vi "SaccadeAnalyser - Main.vi"(8 "error in (no error)":errorcluster, 11 "Data IN":T3={"Impulse Positions"=[{"Start"=5471, "End"=5813, "Impulse Plane"=enum."Yaw", "Impulse Direction +ve?"=FALSE, "Time offset"=0, "Amplitude offset"=0.0}, {"Start"=6974, "End"=7325, "Impulse Plane"=enum."Yaw", "Impulse Direction +ve?"=TRUE, "Time offset"=0, "Amplitude offset"=0.0}, {"Start"=7641, "End"=7980, "Impulse Plane"=enum."Yaw", "Impulse Direction +ve?"=FALSE, "Time offset"=0, "Amplitude offset"=0.0}, {"Start"=9060, "End"=9400, "Impulse Plane"=enum."Yaw", "Impulse Direction +ve?"=FALSE, "Time offset"=0, "Amplitude offset"=0.0}, {"Start"=9938, "End"=10282, "Impulse Plane"=enum."Yaw", "Impulse Direction +ve?"=FALSE, "Time offset"=0, "Amplitude offset"=0.0}, {"Start"=10800, "End"=11142, "Impulse Plane"=enum."Yaw", "Impulse Direction +ve?"=FALSE, "Time offset"=0, "Amplitude offset"=0.0}, {"Start"=11602, "End"=11942, "Impulse Plane"=enum."Yaw", "Impulse Direction +ve?"=TRUE, "Time offset"=0, "Amplitude offset"=0.0}, {"Start"=12449, "End"=12790, "Impulse Plane"=enum."Yaw", "Impulse Direction +ve?"=TRUE, "Time offset"=0, "Amplitude offset"=0.0}, {"Start"=13310, "End"=13653, "Impulse Plane"=enum."Yaw", "Impulse Direction +ve?"=TRUE, "Time offset"=0, "Amplitude offset"=0.0}, {"Start"=14191, "End"=14535, "Impulse Plane"=enum."Yaw", "Impulse Direction +ve?"=TRUE, "Time offset"=0, "Amplitude offset"=0.0}, {"Start"=15040, "End"=15380, "Impulse Plane"=enum."Yaw", "Impulse Direction +ve?"=FALSE, "Time offset"=0, "Amplitude offset"=0.0}, {"Start"=16780, "End"=17124, "Impulse Plane"=enum."Yaw", "Impulse Direction +ve?"=TRUE, "Time offset"=0, "Amplitude offset"=0.0}, {"Start"=17572, "End"=17913, "Impulse Plane"=enum."Yaw", "Impulse Direction +ve?"=FALSE, "Time offset"=0, "Amplitude offset"=0.0}, {"Start"=18369, "End"=18713, "Impulse Plane"=enum."Yaw", "Impulse Direction +ve?"=FALSE, "Time offset"=0, "Amplitude offset"=0.0}, {"Start"=19174, "End"=19519, "Impulse Plane"=enum."Yaw", "Impulse Direction +ve?"=FALSE, "Time offset"=0, "Amplitude offset"=0.0}, {"Start"=19928, "End"=20270, "Impulse Plane"=enum."Yaw", "Impulse Direction +ve?"=TRUE, "Time offset"=0, "Amplitude offset"=0.0}, {"Start"=20762, "End"=21121, "Impulse Plane"=enum."Yaw", "Impulse Direction +ve?"=FALSE, "Time offset"=0, "Amplitude offset"=0.0}, {"Start"=21554, "End"=21888, "Impulse Plane"=enum."Yaw", "Impulse Direction +ve?"=FALSE, "Time offset"=0, "Amplitude offset"=0.0}, {"Start"=22293, "End"=22639, "Impulse Plane"=enum."Yaw", "Impulse Direction +ve?"=TRUE, "Time offset"=0, "Amplitude offset"=0.0}, {"Start"=23109, "End"=23464, "Impulse Plane"=enum."Yaw", "Impulse Direction +ve?"=TRUE, "Time offset"=0, "Amplitude offset"=0.0}, {"Start"=23868, "End"=24215, "Impulse Plane"=enum."Yaw", "Impulse Direction +ve?"=TRUE, "Time offset"=0, "Amplitude offset"=0.0}, {"Start"=24643, "End"=24992, "Impulse Plane"=enum."Yaw", "Impulse Direction +ve?"=FALSE, "Time offset"=0, "Amplitude offset"=0.0}, {"Start"=25685, "End"=26023, "Impulse Plane"=enum."Yaw", "Impulse Direction +ve?"=FALSE, "Time offset"=0, "Amplitude offset"=0.0}, {"Start"=26431, "End"=26768, "Impulse Plane"=enum."Yaw", "Impulse Direction +ve?"=FALSE, "Time offset"=0, "Amplitude offset"=0.0}, {"Start"=27251, "End"=27595, "Impulse Plane"=enum."Yaw", "Impulse Direction +ve?"=FALSE, "Time offset"=0, "Amplitude offset"=0.0}, {"Start"=28832, "End"=29180, "Impulse Plane"=enum."Yaw", "Impulse Direction +ve?"=TRUE, "Time offset"=0, "Amplitude offset"=0.0}, {"Start"=31028, "End"=31383, "Impulse Plane"=enum."LARP", "Impulse Direction +ve?"=FALSE, "Time offset"=0, "Amplitude offset"=0.0}, {"Start"=32603, "End"=32936, "Impulse Plane"=enum."LARP", "Impulse Direction +ve?"=TRUE, "Time offset"=0, "Amplitude offset"=0.0}, {"Start"=33445, "End"=33779, "Impulse Plane"=enum."LARP", "Impulse Direction +ve?"=TRUE, "Time offset"=0, "Amplitude offset"=0.0}, {"Start"=34276, "End"=34629, "Impulse Plane"=enum."LARP", "Impulse Direction +ve?"=FALSE, "Time offset"=0, "Amplitude offset"=0.0}, {"Start"=35114, "End"=35460, "Impulse Plane"=enum."LARP", "Impulse Direction +ve?"=FALSE, "Time offset"=0, "Amplitude offset"=0.0}, {"Start"=35981, "End"=36324, "Impulse Plane"=enum."LARP", "Impulse Direction +ve?"=TRUE, "Time offset"=0, "Amplitude offset"=0.0}, {"Start"=36920, "End"=37249, "Impulse Plane"=enum."LARP", "Impulse Direction +ve?"=TRUE, "Time offset"=0, "Amplitude offset"=0.0}, {"Start"=37988, "End"=38322, "Impulse Plane"=enum."LARP", "Impulse Direction +ve?"=TRUE, "Time offset"=0, "Amplitude offset"=0.0}, {"Start"=38964, "End"=39324, "Impulse Plane"=enum."LARP", "Impulse Direction +ve?"=FALSE, "Time offset"=0, "Amplitude offset"=0.0}, {"Start"=39948, "End"=40284, "Impulse Plane"=enum."LARP", "Impulse Direction +ve?"=TRUE, "Time offset"=0, "Amplitude offset"=0.0}, {"Start"=40958, "End"=41293, "Impulse Plane"=enum."LARP", "Impulse Direction +ve?"=TRUE, "Time offset"=0, "Amplitude offset"=0.0}, {"Start"=41899, "End"=42229, "Impulse Plane"=enum."LARP", "Impulse Direction +ve?"=TRUE, "Time offset"=0, "Amplitude offset"=0.0}, {"Start"=42801, "End"=43154, "Impulse Plane"=enum."LARP", "Impulse Direction +ve?"=FALSE, "Time offset"=0, "Amplitude offset"=0.0}, {"Start"=43641, "End"=43980, "Impulse Plane"=enum."LARP", "Impulse Direction +ve?"=TRUE, "Time offset"=0, "Amplitude offset"=0.0}, {"Start"=44466, "End"=44821, "Impulse Plane"=enum."LARP", "Impulse Direction +ve?"=FALSE, "Time offset"=0, "Amplitude offset"=0.0}, {"Start"=45388, "End"=45722, "Impulse Plane"=enum."LARP", "Impulse Direction +ve?"=TRUE, "Time offset"=0, "Amplitude offset"=0.0}, {"Start"=46149, "End"=46510, "Impulse Plane"=enum."LARP", "Impulse Direction +ve?"=FALSE, "Time offset"=0, "Amplitude offset"=0.0}, {"Start"=47874, "End"=48206, "Impulse Plane"=enum."LARP", "Impulse Direction +ve?"=TRUE, "Time offset"=0, "Amplitude offset"=0.0}, {"Start"=50143, "End"=50479, "Impulse Plane"=enum."RALP", "Impulse Direction +ve?"=TRUE, "Time offset"=0, "Amplitude offset"=0.0}, {"Start"=50976, "End"=51310, "Impulse Plane"=enum."RALP", "Impulse Direction +ve?"=FALSE, "Time offset"=0, "Amplitude offset"=0.0}, {"Start"=51892, "End"=52226, "Impulse Plane"=enum."RALP", "Impulse Direction +ve?"=FALSE, "Time offset"=0, "Amplitude offset"=0.0}, {"Start"=52839, "End"=53171, "Impulse Plane"=enum."RALP", "Impulse Direction +ve?"=FALSE, "Time offset"=0, "Amplitude offset"=0.0}, {"Start"=53676, "End"=54012, "Impulse Plane"=enum."RALP", "Impulse Direction +ve?"=TRUE, "Time offset"=0, "Amplitude offset"=0.0}, {"Start"=54530, "End"=54877, "Impulse Plane"=enum."RALP", "Impulse Direction +ve?"=FALSE, "Time offset"=0, "Amplitude offset"=0.0}, {"Start"=55371, "End"=55711, "Impulse Plane"=enum."RALP", "Impulse Direction +ve?"=TRUE, "Time offset"=0, "Amplitude offset"=0.0}, {"Start"=56153, "End"=56482, "Impulse Plane"=enum."RALP", "Impulse Direction +ve?"=FALSE, "Time offset"=0, "Amplitude offset"=0.0}, {"Start"=57053, "End"=57390, "Impulse Plane"=enum."RALP", "Impulse Direction +ve?"=FALSE, "Time offset"=0, "Amplitude offset"=0.0}, {"Start"=57954, "End"=58292, "Impulse Plane"=enum."RALP", "Impulse Direction +ve?"=FALSE, "Time offset"=0, "Amplitude offset"=0.0}, {"Start"=58794, "End"=59130, "Impulse Plane"=enum."RALP", "Impulse Direction +ve?"=TRUE, "Time offset"=0, "Amplitude offset"=0.0}, {"Start"=59587, "End"=59931, "Impulse Plane"=enum."RALP", "Impulse Direction +ve?"=TRUE, "Time offset"=0, "Amplitude offset"=0.0}, {"Start"=60399, "End"=60744, "Impulse Plane"=enum."RALP", "Impulse Direction +ve?"=FALSE, "Time offset"=0, "Amplitude offset"=0.0}, {"Start"=61218, "End"=61559, "Impulse Plane"=enum."RALP", "Impulse Direction +ve?"=FALSE, "Time offset"=0, "Amplitude offset"=0.0}, {"Start"=62100, "End"=62442, "Impulse Plane"=enum."RALP", "Impulse Direction +ve?"=FALSE, "Time offset"=0, "Amplitude offset"=0.0}, {"Start"=62989, "End"=63322, "Impulse Plane"=enum."RALP", "Impulse Direction +ve?"=FALSE, "Time offset"=0, "Amplitude offset"=0.0}, {"Start"=63787, "End"=64136, "Impulse Plane"=enum."RALP", "Impulse Direction +ve?"=TRUE, "Time offset"=0, "Amplitude offset"=0.0}, {"Start"=64603, "End"=64953, "Impulse Plane"=enum."RALP", "Impulse Direction +ve?"=FALSE, "Time offset"=0, "Amplitude offset"=0.0}, {"Start"=65462, "End"=65795, "Impulse Plane"=enum."RALP", "Impulse Direction +ve?"=FALSE, "Time offset"=0, "Amplitude offset"=0.0}, {"Start"=66308, "End"=66645, "Impulse Plane"=enum."RALP", "Impulse Direction +ve?"=FALSE, "Time offset"=0, "Amplitude offset"=0.0}, {"Start"=67052, "End"=67402, "Impulse Plane"=enum."RALP", "Impulse Direction +ve?"=TRUE, "Time offset"=0, "Amplitude offset"=0.0}], "No. Imp"=15, "Parameter Time Series"=[{"time offset"=0.0, "Offset"=0.0, "Gain"=1.0, "inverse"=FALSE, "filter data"=FALSE, "dots"=FALSE, "interpolate"=FALSE, "List 1"=5, "Color Box"=6618880, "Boolean"=TRUE}, {"time offset"=0.0, "Offset"=0.0, "Gain"=1.0, "inverse"=FALSE, "filter data"=FALSE, "dots"=FALSE, "interpolate"=FALSE, "List 1"=6, "Color Box"=6618880, "Boolean"=FALSE}, {"time offset"=0.0, "Offset"=0.0, "Gain"=1.0, "inverse"=FALSE, "filter data"=FALSE, "dots"=FALSE, "interpolate"=FALSE, "List 1"=7, "Color Box"=6618880, "Boolean"=FALSE}, {"time offset"=0.0, "Offset"=0.0, "Gain"=1.0, "inverse"=FALSE, "filter data"=FALSE, "dots"=FALSE, "interpolate"=FALSE, "List 1"=13, "Color Box"=16777224, "Boolean"=TRUE}, {"time offset"=0.0, "Offset"=0.0, "Gain"=1.0, "inverse"=FALSE, "filter data"=FALSE, "dots"=FALSE, "interpolate"=FALSE, "List 1"=14, "Color Box"=16777224, "Boolean"=FALSE}, {"time offset"=0.0, "Offset"=0.0, "Gain"=1.0, "inverse"=FALSE, "filter data"=FALSE, "dots"=FALSE, "interpolate"=FALSE, "List 1"=15, "Color Box"=16777224, "Boolean"=FALSE}], "Parameter Impuls Series"=[{"Color"=6618880, "Visible"=TRUE, "Channel"=1, "Invert"=FALSE, "Desaccade"=FALSE, "Offset"=0.0, "Gain"=1.0}, {"Color"=6618880, "Visible"=FALSE, "Channel"=6, "Invert"=FALSE, "Desaccade"=FALSE, "Offset"=0.0, "Gain"=1.0}, {"Color"=6618880, "Visible"=FALSE, "Channel"=7, "Invert"=FALSE, "Desaccade"=FALSE, "Offset"=0.0, "Gain"=1.0}, {"Color"=16777224, "Visible"=TRUE, "Channel"=13, "Invert"=FALSE, "Desaccade"=FALSE, "Offset"=0.0, "Gain"=1.0}, {"Color"=16777224, "Visible"=FALSE, "Channel"=14, "Invert"=FALSE, "Desaccade"=FALSE, "Offset"=0.0, "Gain"=1.0}, {"Color"=16777224, "Visible"=FALSE, "Channel"=15, "Invert"=FALSE, "Desaccade"=FALSE, "Offset"=0.0, "Gain"=1.0}], "Experiment Parameters"={"Freq"=0.0, "Vel"=0, "Acc"=0, "Stimulus"="Head Impulse"}, "Autosort File"=refnum, "Data File"={"Data Channels"=array34x71049[2415666 elements], "Sample Rate"=500, "Channel List"=["Hz Position-in-Head", "Hz Velocity-in-Head", "Hy Position-in-Head", "Hy Velocity-in-Head", "Hx Position-in-Head", "Hx Velocity-in-Head", "Hl Velocity-in-Head", "Hr Velocity-in-Head", "Lx Position-in-Head", "Ly Position-in-Head", "Lz Position-in-Head", "Lx Velocity-in-Head", "Ly Velocity-in-Head", "Lz Velocity-in-Head", "Ll Velocity-in-Head", "Lr Velocity-in-Head", "Rx Position-in-Head", "Ry Position-in-Head", "Rz Position-in-Head", "Rx Velocity-in-Head", "Ry Velocity-in-Head", "Rz Velocity-in-Head", "Rl Velocity-in-Head", "Rr Velocity-in-Head", "Target on/off", "aux input 1", "aux input 2", " ", "", "", "", "Target Hor", "Target Ver", ""]}, "Experiment data path"=path "C:/Users/w.figtree/Desktop/Coils Data/3", "Image data path"=path "/Macintosh HD/Users/patrick/Studium/Diploma Thesis/Data Analysis", "LVS data path"=path "/Macintosh HD/Users/patrick/Studium/Diploma Thesis/Data Analysis", "Raw copy path"=path "/Macintosh HD/Users/patrick/Studium/Diploma Thesis/Data Analysis", "filename"="passive_lvs.lvs", "desaccading parameters"={"Tolerance"=3, "Acc Range"=7000.0, "Sample Rate"=500, "Impulse Plane 2"=enum."Yaw", "Impulse dir"=FALSE}, "Experiment Parameters 2"={"Subject"="SE Trial Short Term", "Strain"="", "Rotation plane"="", "Experimenter"=" ", "Trial"=0.0, "Time"=0.0}, "Excel"={"Excel._Application"=refnum, "Use Excel"=TRUE, "Worksheet SINE"=refnum, "Row SINE"=0, "Worksheet TRANS"=refnum, "Row TRANS"=0}, "Session Config File"=refnum, "Autosort Parameter Set"=4, "EMA Version"="EMA 2016a", "desacc "={"Threshold 1 [Acc]"=7000.0, "Threshold 2 [% of TH1]"=60, "tolerance"=3, "Search WD "=0.1, " always use TH2"=FALSE, "Range"=3.0, "Max time"=120.0, "Min time"=20.0, "Velocity Threshold"=150}, "Cycle Nr for Saccades"={"POS"=0, "NEG"=0}, "calibration name"="u_calibration_1_p00001s001_calib.mat", "Excel"=refnum} {"Parameter Time Series"."time offset" format="%.3f"; "Parameter Time Series"."Gain" format="%.1f"; "Parameter Time Series"."Offset" format="%.1f"; "Parameter Time Series"."List 1" items=["Motor-Pos", "Motor-Vel", "Lx Position-in-Head", "Ly Position-in-Head", "Lz Position-in-Head", "Lx Velocity-in-Head", "Ly Velocity-in-Head", "Lz Velocity-in-Head", "Ll Velocity-in-Head", "Lr Velocity-in-Head", "Lx Accel-in-Head", "Ly Accel-in-Head", "Lz Accel-in-Head", "Rx Position-in-Head", "Ry Position-in-Head", "Rz Position-in-Head", "Rx Velocity-in-Head", "Ry Velocity-in-Head", "Rz Velocity-in-Head", "Rl Velocity-in-Head", "Rr Velocity-in-Head", "Rx Accel-in-Head", "Ry Accel-in-Head", "Rz Accel-in-Head", "Global Trigger", "", "", ""]; "Parameter Impuls Series"."Gain" format="%.1f"; "Parameter Impuls Series"."Offset" format="%.1f"}) -> (0 "error out":errorcluster, 3 "Data OUT":T3={"Impulse Positions"=[{"Start"=5471, "End"=5813, "Impulse Plane"=enum."Yaw", "Impulse Direction +ve?"=FALSE, "Time offset"=0, "Amplitude offset"=0.0}, {"Start"=6974, "End"=7325, "Impulse Plane"=enum."Yaw", "Impulse Direction +ve?"=TRUE, "Time offset"=0, "Amplitude offset"=0.0}, {"Start"=7641, "End"=7980, "Impulse Plane"=enum."Yaw", "Impulse Direction +ve?"=FALSE, "Time offset"=0, "Amplitude offset"=0.0}, {"Start"=9060, "End"=9400, "Impulse Plane"=enum."Yaw", "Impulse Direction +ve?"=FALSE, "Time offset"=0, "Amplitude offset"=0.0}, {"Start"=9938, "End"=10282, "Impulse Plane"=enum."Yaw", "Impulse Direction +ve?"=FALSE, "Time offset"=0, "Amplitude offset"=0.0}, {"Start"=10800, "End"=11142, "Impulse Plane"=enum."Yaw", "Impulse Direction +ve?"=FALSE, "Time offset"=0, "Amplitude offset"=0.0}, {"Start"=11602, "End"=11942, "Impulse Plane"=enum."Yaw", "Impulse Direction +ve?"=TRUE, "Time offset"=0, "Amplitude offset"=0.0}, {"Start"=12449, "End"=12790, "Impulse Plane"=enum."Yaw", "Impulse Direction +ve?"=TRUE, "Time offset"=0, "Amplitude offset"=0.0}, {"Start"=13310, "End"=13653, "Impulse Plane"=enum."Yaw", "Impulse Direction +ve?"=TRUE, "Time offset"=0, "Amplitude offset"=0.0}, {"Start"=14191, "End"=14535, "Impulse Plane"=enum."Yaw", "Impulse Direction +ve?"=TRUE, "Time offset"=0, "Amplitude offset"=0.0}, {"Start"=15040, "End"=15380, "Impulse Plane"=enum."Yaw", "Impulse Direction +ve?"=FALSE, "Time offset"=0, "Amplitude offset"=0.0}, {"Start"=16780, "End"=17124, "Impulse Plane"=enum."Yaw", "Impulse Direction +ve?"=TRUE, "Time offset"=0, "Amplitude offset"=0.0}, {"Start"=17572, "End"=17913, "Impulse Plane"=enum."Yaw", "Impulse Direction +ve?"=FALSE, "Time offset"=0, "Amplitude offset"=0.0}, {"Start"=18369, "End"=18713, "Impulse Plane"=enum."Yaw", "Impulse Direction +ve?"=FALSE, "Time offset"=0, "Amplitude offset"=0.0}, {"Start"=19174, "End"=19519, "Impulse Plane"=enum."Yaw", "Impulse Direction +ve?"=FALSE, "Time offset"=0, "Amplitude offset"=0.0}, {"Start"=19928, "End"=20270, "Impulse Plane"=enum."Yaw", "Impulse Direction +ve?"=TRUE, "Time offset"=0, "Amplitude offset"=0.0}, {"Start"=20762, "End"=21121, "Impulse Plane"=enum."Yaw", "Impulse Direction +ve?"=FALSE, "Time offset"=0, "Amplitude offset"=0.0}, {"Start"=21554, "End"=21888, "Impulse Plane"=enum."Yaw", "Impulse Direction +ve?"=FALSE, "Time offset"=0, "Amplitude offset"=0.0}, {"Start"=22293, "End"=22639, "Impulse Plane"=enum."Yaw", "Impulse Direction +ve?"=TRUE, "Time offset"=0, "Amplitude offset"=0.0}, {"Start"=23109, "End"=23464, "Impulse Plane"=enum."Yaw", "Impulse Direction +ve?"=TRUE, "Time offset"=0, "Amplitude offset"=0.0}, {"Start"=23868, "End"=24215, "Impulse Plane"=enum."Yaw", "Impulse Direction +ve?"=TRUE, "Time offset"=0, "Amplitude offset"=0.0}, {"Start"=24643, "End"=24992, "Impulse Plane"=enum."Yaw", "Impulse Direction +ve?"=FALSE, "Time offset"=0, "Amplitude offset"=0.0}, {"Start"=25685, "End"=26023, "Impulse Plane"=enum."Yaw", "Impulse Direction +ve?"=FALSE, "Time offset"=0, "Amplitude offset"=0.0}, {"Start"=26431, "End"=26768, "Impulse Plane"=enum."Yaw", "Impulse Direction +ve?"=FALSE, "Time offset"=0, "Amplitude offset"=0.0}, {"Start"=27251, "End"=27595, "Impulse Plane"=enum."Yaw", "Impulse Direction +ve?"=FALSE, "Time offset"=0, "Amplitude offset"=0.0}, {"Start"=28832, "End"=29180, "Impulse Plane"=enum."Yaw", "Impulse Direction +ve?"=TRUE, "Time offset"=0, "Amplitude offset"=0.0}, {"Start"=31028, "End"=31383, "Impulse Plane"=enum."LARP", "Impulse Direction +ve?"=FALSE, "Time offset"=0, "Amplitude offset"=0.0}, {"Start"=32603, "End"=32936, "Impulse Plane"=enum."LARP", "Impulse Direction +ve?"=TRUE, "Time offset"=0, "Amplitude offset"=0.0}, {"Start"=33445, "End"=33779, "Impulse Plane"=enum."LARP", "Impulse Direction +ve?"=TRUE, "Time offset"=0, "Amplitude offset"=0.0}, {"Start"=34276, "End"=34629, "Impulse Plane"=enum."LARP", "Impulse Direction +ve?"=FALSE, "Time offset"=0, "Amplitude offset"=0.0}, {"Start"=35114, "End"=35460, "Impulse Plane"=enum."LARP", "Impulse Direction +ve?"=FALSE, "Time offset"=0, "Amplitude offset"=0.0}, {"Start"=35981, "End"=36324, "Impulse Plane"=enum."LARP", "Impulse Direction +ve?"=TRUE, "Time offset"=0, "Amplitude offset"=0.0}, {"Start"=36920, "End"=37249, "Impulse Plane"=enum."LARP", "Impulse Direction +ve?"=TRUE, "Time offset"=0, "Amplitude offset"=0.0}, {"Start"=37988, "End"=38322, "Impulse Plane"=enum."LARP", "Impulse Direction +ve?"=TRUE, "Time offset"=0, "Amplitude offset"=0.0}, {"Start"=38964, "End"=39324, "Impulse Plane"=enum."LARP", "Impulse Direction +ve?"=FALSE, "Time offset"=0, "Amplitude offset"=0.0}, {"Start"=39948, "End"=40284, "Impulse Plane"=enum."LARP", "Impulse Direction +ve?"=TRUE, "Time offset"=0, "Amplitude offset"=0.0}, {"Start"=40958, "End"=41293, "Impulse Plane"=enum."LARP", "Impulse Direction +ve?"=TRUE, "Time offset"=0, "Amplitude offset"=0.0}, {"Start"=41899, "End"=42229, "Impulse Plane"=enum."LARP", "Impulse Direction +ve?"=TRUE, "Time offset"=0, "Amplitude offset"=0.0}, {"Start"=42801, "End"=43154, "Impulse Plane"=enum."LARP", "Impulse Direction +ve?"=FALSE, "Time offset"=0, "Amplitude offset"=0.0}, {"Start"=43641, "End"=43980, "Impulse Plane"=enum."LARP", "Impulse Direction +ve?"=TRUE, "Time offset"=0, "Amplitude offset"=0.0}, {"Start"=44466, "End"=44821, "Impulse Plane"=enum."LARP", "Impulse Direction +ve?"=FALSE, "Time offset"=0, "Amplitude offset"=0.0}, {"Start"=45388, "End"=45722, "Impulse Plane"=enum."LARP", "Impulse Direction +ve?"=TRUE, "Time offset"=0, "Amplitude offset"=0.0}, {"Start"=46149, "End"=46510, "Impulse Plane"=enum."LARP", "Impulse Direction +ve?"=FALSE, "Time offset"=0, "Amplitude offset"=0.0}, {"Start"=47874, "End"=48206, "Impulse Plane"=enum."LARP", "Impulse Direction +ve?"=TRUE, "Time offset"=0, "Amplitude offset"=0.0}, {"Start"=50143, "End"=50479, "Impulse Plane"=enum."RALP", "Impulse Direction +ve?"=TRUE, "Time offset"=0, "Amplitude offset"=0.0}, {"Start"=50976, "End"=51310, "Impulse Plane"=enum."RALP", "Impulse Direction +ve?"=FALSE, "Time offset"=0, "Amplitude offset"=0.0}, {"Start"=51892, "End"=52226, "Impulse Plane"=enum."RALP", "Impulse Direction +ve?"=FALSE, "Time offset"=0, "Amplitude offset"=0.0}, {"Start"=52839, "End"=53171, "Impulse Plane"=enum."RALP", "Impulse Direction +ve?"=FALSE, "Time offset"=0, "Amplitude offset"=0.0}, {"Start"=53676, "End"=54012, "Impulse Plane"=enum."RALP", "Impulse Direction +ve?"=TRUE, "Time offset"=0, "Amplitude offset"=0.0}, {"Start"=54530, "End"=54877, "Impulse Plane"=enum."RALP", "Impulse Direction +ve?"=FALSE, "Time offset"=0, "Amplitude offset"=0.0}, {"Start"=55371, "End"=55711, "Impulse Plane"=enum."RALP", "Impulse Direction +ve?"=TRUE, "Time offset"=0, "Amplitude offset"=0.0}, {"Start" (continued)
52.608407400318306, 68.06098679809003, 80.42943215585183, 88.0864760597265, 89.99891509546197, 85.90799751985459, 76.36544752990858, 62.62091186359373, 46.38143453236263, 29.50492183788016, 13.707859867290857, 0.3310928457604554, -9.810012583460072, -16.45442202598098, -19.82247119153461, -20.483452553608764, -19.193953324369854, -16.74774940350339, -13.849446600754366, -11.037569111752362, -8.669405751207828, -6.917292102316395, -5.789797050590641, -5.190164981316045, -4.962518505347841, -4.93187469016212, -4.9320919709982025, -4.837167605556909, -4.587847044554708, -4.179208179540813, -3.659763768094379, -3.1208090278845084, -2.653103860344153, -2.3271525568125213, -2.1861172612544255, -2.233842916743079, -2.446189563900692, -2.777356551203642, -3.1729115127205407, -3.593585048501322, -4.014858546360711, -4.426484406643328, -4.830051913071344, -5.225505364127684, -5.604699028522771, -5.955284071910426, -6.265984392521009, -6.532840549008947, -6.76267990262583, -6.974346991783459, -7.191231058870271, -7.441351509284662, -7.752342029197125, -8.138375237447635, -8.601195262840081, -9.123078516960476, -9.673239943518213, -10.219145635835941, -10.716542542217685, -11.114227594642026, -11.370082247719761, -11.451375205364059, -11.348722192681933, -11.089585339730856, -10.727486236031975, -10.343142553232035, -10.037654243821347, -9.907641710473694, -10.028124243024223, -10.440559585131421, -11.147679111533204, -12.104742918852578, -13.216616186504224, -14.363595848676741, -15.431203656896052, -16.31897411242039, -16.94639318528374, -17.271721118269923, -17.301470159658848, -17.08278383403612, -16.6966662886884, -16.245543532611645, -15.834108566842296, -15.559718461265135, -15.498960178465857]}, {[0.0, 2.0, 4.0, 6.0, 8.0, 10.0, 12.0, 14.0, 16.0, 18.000000000000004, 20.0, 22.0, 24.0, 26.000000000000004, 28.0, 30.0, 32.0, 34.0, 36.00000000000001, 38.0, 40.0, 42.0, 44.0, 46.0, 48.0, 50.0, 52.00000000000001, 54.0, 56.0, 58.0, 60.0, 62.0, 64.0, 66.0, 68.0, 70.0, 72.00000000000001, 74.0, 76.0, 78.0, 80.0, 82.0, 84.0, 86.0, 88.0, 90.0, 92.0, 94.0, 96.0, 98.0, 100.0, 102.00000000000001, 104.00000000000001, 106.0, 108.0, 110.0, 112.0, 114.0, 116.0, 118.00000000000001, 120.0, 122.0, 124.0, 126.0, 128.0, 130.0, 132.0, 134.0, 136.0, 138.0, 140.0, 142.00000000000003, 144.00000000000003, 146.0, 148.0, 150.0, 152.0, 154.0, 156.0, 158.0, 160.0, 162.0, 164.0, 166.0, 168.0, 170.0, 172.0, 174.00000000000003, 176.0, 178.0, 180.0, 182.0, 184.0, 186.0, 188.0, 190.0, 192.0, 194.0, 196.0, 198.0, 200.0, 202.0, 204.00000000000003, 206.00000000000003, 208.00000000000003, 210.0, 212.0, 214.0, 216.0, 218.0, 220.0, 222.0, 224.0, 226.0, 228.0, 230.0, 232.0, 234.0, 236.00000000000003, 238.00000000000003, 240.0, 242.0, 244.0, 246.0, 248.0, 250.0, 252.0, 254.0, 256.0, 258.0, 260.0, 262.0, 264.0, 266.0, 268.0, 270.0, 272.0, 274.0, 276.0, 278.0, 280.0, 282.0, 284.00000000000006, 286.00000000000006, 288.00000000000006, 290.0, 292.0, 294.0, 296.0, 298.0, 300.0, 302.0, 304.0, 306.0, 308.0, 310.0, 312.0, 314.0, 316.0, 318.0, 320.0, 322.0, 324.0, 326.0, 328.0, 330.0, 332.0, 334.0, 336.0, 338.0, 340.0, 342.0, 344.0, 346.00000000000006, 348.00000000000006, 350.00000000000006, 352.0, 354.0, 356.0, 358.0, 360.0, 362.0, 364.0, 366.0, 368.0, 370.0, 372.0, 374.0, 376.0, 378.0, 380.0, 382.0, 384.0, 386.0, 388.0, 390.0, 392.0, 394.0, 396.0, 398.0, 400.0, 402.0, 404.0, 406.0, 408.00000000000006, 410.00000000000006, 412.00000000000006, 414.00000000000006, 416.00000000000006, 418.0, 420.0, 422.0, 424.0, 426.0, 428.0, 430.0, 432.0, 434.0, 436.0, 438.0, 440.0, 442.0, 444.0, 446.0, 448.0, 450.0, 452.0, 454.0, 456.0, 458.0, 460.0, 462.0, 464.0, 466.0, 468.0, 470.00000000000006, 472.00000000000006, 474.00000000000006, 476.00000000000006, 478.00000000000006, 480.0, 482.0, 484.0, 486.0, 488.0, 490.0, 492.0, 494.0, 496.0, 498.0, 500.0, 502.0, 504.0, 506.0, 508.0, 510.0, 512.0, 514.0, 516.0, 518.0, 520.0, 522.0, 524.0, 526.0, 528.0, 530.0, 532.0, 534.0, 536.0, 538.0, 540.0, 542.0, 544.0, 546.0, 548.0, 550.0, 552.0, 554.0, 556.0, 558.0, 560.0, 562.0, 564.0, 566.0000000000001, 568.0000000000001, 570.0000000000001, 572.0000000000001, 574.0000000000001, 576.0000000000001, 578.0, 580.0, 582.0, 584.0, 586.0, 588.0, 590.0, 592.0, 594.0, 596.0, 598.0, 600.0, 602.0, 604.0, 606.0, 608.0, 610.0, 612.0, 614.0, 616.0, 618.0, 620.0, 622.0, 624.0, 626.0, 628.0, 630.0, 632.0, 634.0, 636.0, 638.0, 640.0, 642.0, 644.0, 646.0, 648.0, 650.0, 652.0, 654.0, 656.0, 658.0, 660.0, 662.0, 664.0, 666.0, 668.0], [-0.2084737640001224, -0.21061254423196019, -0.19974340239986255, -0.1814526364220792, -0.15950621992842695, -0.13869454883876742, -0.1230229953936619, -0.11265601439465467, -0.10478068393938789, -0.08868410182101516, -0.04651793076238242, 0.04375652472078573, 0.20699981625307806, 0.4630259746711778, 0.8167071478046634, 1.249476497931788, 1.7158757069759787, 2.148078458394064, 2.4679527713133727, 2.605475170750913, 2.517129266334929, 2.204076444324693, 1.723582173586595, 1.1780633063446757, 0.6932523935605728, 0.39190365772674873, 0.36316476090271355, 0.6373868501280575, 1.1716341468731537, 1.8542801136034845, 2.5294296065937605, 3.0333677147052893, 3.2353202176928115, 3.072554893536261, 2.568412986254921, 1.8284693921231296, 1.0173284987993005, 0.319471626398907, -0.10572049000990091, -0.1618122134221225, 0.1624566895403241, 0.7891090567724359, 1.576050899857925, 2.3578045708496624, 2.9725118541262665, 3.291856565626881, 3.2561829028184293, 2.8868512950404415, 2.2656505875726585, 1.5088004738797285, 0.7449184275149427, 0.0888948481514934, -0.3778537505248051, -0.6153274128319215, -0.6271601340363961, -0.455205322855745, -0.16230527407613415, 0.17313725908850575, 0.4732306012970348, 0.6792232665989548, 0.7452703193414447, 0.6399322732108803, 0.3518492398694276, -0.10965738361630661, -0.716763835932134, -1.432468908324777, -2.2171396049387964, -3.0298284691754356, -3.840267049354215, -4.639809300711624, -5.439157523515876, -6.271967711479519, -7.18995317163518, -8.25313765393062, -9.522747383362622, -11.047226568583898, -12.858240051696878, -14.966387351509574, -17.362286476817644, -20.024081485551548, -22.91926202136785, -26.01774958679112, -29.305849031733096, -32.78186481781676, -36.457227063732205, -40.35964473833927, -44.51334065936565, -48.92764087528358, -53.591641734355996, -58.46483429775378, -63.47962090894122, -68.5545913643943, -73.60762377558018, -78.5664986699027, -83.38683304180586, -88.06213476697582, -92.61554589462526, -97.07737768506577, -101.47278024524172, -105.81704377266682, -110.09651253699154, -114.2627035739459, -118.24660811311482, -121.96750598733041, -125.34737086154962, -128.32701096818022, -130.8713821879744, -132.9742608220829, -134.6511985155471, -135.9377463748218, -136.88254905466255, -137.53225496837416, -137.92883917338443, -138.1004332018286, -138.0547295805257, -137.7822752357644, -137.25823564259645, -136.43624394768, -135.26009007675424, -133.68504834005822, -131.67503683545578, -129.21239879273423, -126.31496987566545, -123.02992432867316, -119.42662603331583, -115.58493896478993, -111.58035425385465, -107.47140704418365, -103.28456891587382, -99.01030341243388, -94.60778573645524, -90.02287685553279, -85.21465969682528, -80.16515023394788, -74.89235717152984, -69.46633382179459, -63.988964393102904, -58.57246381234703, -53.33346565335498, -48.36457788040865, -43.716496037766944, -39.40476353500591, -35.40559331498966, -31.667477528327385, -28.13468472959024, -24.759920204946503, -21.518151545705557, -18.406017738139635, -15.439347619240051, -12.654467099258708, -10.09194617547714, -7.774397556953381, -5.705376259087573, -3.872295523002112, -2.240851888552726, -0.7669274233185266, 0.5840961633948889, 1.827583172760238, 2.951473953311094, 3.9027615305468775, 4.60333887313916, 4.981833760650325, 4.983720475139977, 4.593660156925323, 3.8574255841263114, 2.8740801218048437, 1.7840413317484587, 0.7520745682651158, -0.06867418369201594, -0.5704650490739693, -0.7148528403732115, -0.5367098293553876, -0.12623205069174626, 0.397721777004826, 0.9123004379504209, 1.3229343997828682, 1.5926915922407034, 1.7398163810383567, 1.830045623817825, 1.9600722237695143, 2.2245315967506016, 2.6915390877746463, 3.38930839852143, 4.2963754755709544, 5.351352806866268, 6.468714941199869, 7.558863565059841, 8.557435143222357, 9.424176367037068, 10.143380548437653, 10.728077252221851, 11.206782621949968, 11.612745771770005, 11.96941118817539, 12.282297221521992, 12.545902968163706, 12.75479662246264, 12.907280046975862, 13.002946881268697, 13.048070216870075, 13.05658923212351, 13.042999977014594, 13.009977061471465, 12.94245475766868, 12.81890063153454, 12.609765366914898, 12.278184473350246, 11.797051098842251, 11.163225835782933, 10.393011826590396, 9.522113727171078, 8.615425896177715, 7.745082529904571, 6.979041714673084, 6.3806875710243816, 5.987280438025684, 5.808451827363265, 5.825830619890626, 5.988734979148465, 6.235029270749025, 6.497307570326141, 6.708414886955869, 6.825333412494453, 6.838975547429279, 6.77119240758477, 6.665661088127153, 6.5825795781284775, 6.585157617597242, 6.7190404467055025, 7.0047361683227125, 7.427956588477651, 7.936103473475136, 8.457973857413847, 8.91663794274779, 9.24592372051221, 9.41299003052989, 9.42128335760351, 9.313816088053846, 9.160197824100333, 9.03422460503209, 9.00332035204722, 9.110964558431714, 9.356477246081301, 9.697905817665067, 10.068707122553423, 10.392118640423174, 10.603580854248928, 10.666148434748134, 10.571062625263746, 10.337853733632475, 10.006528955246454, 9.620364236757855, 9.212151855400645, 8.797154334020405, 8.379159772372343, 7.957296849470608, 7.528419211992924, 7.097575516571727, 6.685985131118928, 6.319061420298434, 6.012401551740286, 5.772644540633117, 5.591239306405097, 5.441314182743255, 5.288411099253823, 5.102450883850739, 4.871976546334581, 4.60251734588017, 4.311090632023168, 4.028743938240488, 3.7830247655802403, 3.5796176831348223, 3.4054550735736697, 3.2383203495831623, 3.056274327318306, 2.8384458855153802, 2.577574401150361, 2.294924077968048, 2.0263453687840567, 1.8160246303966208, 1.7097372924102583, 1.7288918176049108, 1.8693764818405159, 2.109389815808658, 2.41175024674149, 2.742929315582983, 3.0765384739198836, 3.398505542181912, 3.712913054967018, 4.033330189618671, 4.378551273101138, 4.758520962222116, 5.163138467507516, 5.569135136295238, 5.953447283858051, 6.298919732057598, 6.598321475833523, 6.86094942777693, 7.1113291647146575, 7.376361618381718, 7.677069880203424, 8.023229526040426, 8.410567550278042, 8.820913458363085, 9.225801583554672, 9.601658109813517, 9.941323778543545, 10.250891695805471, 10.543402599193524, 10.836488737807839, 11.138908355314491, 11.450052897014324, 11.765042086453594, 12.065061454472708, 12.32961679974079, 12.548835715429114, 12.721987803630839, 12.862685610761266, 13.001440143935076, 13.183667301799584, 13.452412660624564, 13.826963043086014, 14.304812323329203, 14.86791542852336, 15.473438446474717, 16.051514909725263, 16.526779204466816, 16.84258461113391, 16.969078970918382, 16.909195783143538, 16.704519827280293, 16.42693162234456, 16.167802833706965, 16.019740754652858]}, {[0.0, 2.0, 4.0, 6.0, 8.0, 10.0, 12.0, 14.0, 16.0, 18.000000000000004, 20.0, 22.0, 24.0, 26.000000000000004, 28.0, 30.0, 32.0, 34.0, 36.00000000000001, 38.0, 40.0, 42.0, 44.0, 46.0, 48.0, 50.0, 52.00000000000001, 54.0, 56.0, 58.0, 60.0, 62.0, 64.0, 66.0, 68.0, 70.0, 72.00000000000001, 74.0, 76.0, 78.0, 80.0, 82.0, 84.0, 86.0, 88.0, 90.0, 92.0, 94.0, 96.0, 98.0, 100.0, 102.00000000000001, 104.00000000000001, 106.0, 108.0, 110.0, 112.0, 114.0, 116.0, 118.00000000000001, 120.0, 122.0, 124.0, 126.0, 128.0, 130.0, 132.0, 134.0, 136.0, 138.0, 140.0, 142.00000000000003, 144.00000000000003, 146.0, 148.0, 150.0, 152.0, 154.0, 156.0, 158.0, 160.0, 162.0, 164.0, 166.0, 168.0, 170.0, 172.0, 174.00000000000003, 176.0, 178.0, 180.0, 182.0, 184.0, 186.0, 188.0, 190.0, 192.0, 194.0, 196.0, 198.0, 200.0, 202.0, 204.00000000000003, 206.00000000000003, 208.00000000000003, 210.0, 212.0, 214.0, 216.0, 218.0, 220.0, 222.0, 224.0, 226.0, 228.0, 230.0, 232.0, 234.0, 236.00000000000003, 238.00000000000003, 240.0, 242.0, 244.0, 246.0, 248.0, 250.0, 252.0, 254.0, 256.0, 258.0, 260.0, 262.0, 264.0, 266.0, 268.0, 270.0, 272.0, 274.0, 276.0, 278.0, 280.0, 282.0, 284.00000000000006, 286.00000000000006, 288.00000000000006, 290.0, 292.0, 294.0, 296.0, 298.0, 300.0, 302.0, 304.0, 306.0, 308.0, 310.0, 312.0, 314.0, 316.0, 318.0, 320.0, 322.0, 324.0, 326.0, 328.0, 330.0, 332.0, 334.0, 336.0, 338.0, 340.0, 342.0, 344.0, 346.00000000000006, 348.00000000000006, 350.00000000000006, 352.0, 354.0, 356.0, 358.0, 360.0, 362.0, 364.0, 366.0, 368.0, 370.0, 372.0, 374.0, 376.0, 378.0, 380.0, 382.0, 384.0, 386.0, 388.0, 390.0, 392.0, 394.0, 396.0, 398.0, 400.0, 402.0, 404.0, 406.0, 408.00000000000006, 410.00000000000006, 412.00000000000006, 414.00000000000006, 416.00000000000006, 418.0, 420.0, 422.0, 424.0, 426.0, 428.0, 430.0, 432.0, 434.0, 436.0, 438.0, 440.0, 442.0, 444.0, 446.0, 448.0, 450.0, 452.0, 454.0, 456.0, 458.0, 460.0, 462.0, 464.0, 466.0, 468.0, 470.00000000000006, 472.00000000000006, 474.00000000000006, 476.00000000000006, 478.00000000000006, 480.0, 482.0, 484.0, 486.0, 488.0, 490.0, 492.0, 494.0, 496.0, 498.0, 500.0, 502.0, 504.0, 506.0, 508.0, 510.0, 512.0, 514.0, 516.0, 518.0, 520.0, 522.0, 524.0, 526.0, 528.0, 530.0, 532.0, 534.0, 536.0, 538.0, 540.0, 542.0, 544.0, 546.0, 548.0, 550.0, 552.0, 554.0, 556.0, 558.0, 560.0, 562.0, 564.0, 566.0000000000001, 568.0000000000001, 570.0000000000001, 572.0000000000001, 574.0000000000001, 576.0000000000001, 578.0, 580.0, 582.0, 584.0, 586.0, 588.0, 590.0, 592.0, 594.0, 596.0, 598.0, 600.0, 602.0, 604.0, 606.0, 608.0, 610.0, 612.0, 614.0, 616.0, 618.0, 620.0, 622.0, 624.0, 626.0, 628.0, 630.0, 632.0, 634.0, 636.0, 638.0, 640.0, 642.0, 644.0, 646.0, 648.0, 650.0, 652.0, 654.0, 656.0, 658.0, 660.0, 662.0, 664.0, 666.0, 668.0], [0.0918796302143563, 0.03051187266610711, -0.1611957083582869, -0.4704791476531671, -0.8523728519677629, -1.2440649764217149, -1.576434015521139, -1.7796701196194302, -1.7938953581603494, -1.5795532815103304, -1.1244295998384572, -0.45198178461689054, 0.37868924990104347, 1.2845638853841521, 2.1583744757768404, 2.8795083731687825, 3.346162681330089, 3.4904807525699173, 3.287365477540023, 2.76654653904259, 2.0051361995272536, 1.1137776184743124, 0.22312181849178003, -0.5433245412302696, -1.097857981316337, -1.3942687786685717, -1.4203799265812567, -1.2069131330353375, -0.8121129113797165, -0.29213689959068834, 0.3019719271273712, 0.928268615852843, 1.5514165823021486, 2.1282052538836247, 2.6087872333497035, 2.9363407794125846, 3.0422638724853943, 2.872994829020696, 2.41253814956635, 1.6878100685884903, 0.773479470659515, -0.20749246660970044, -1.099066041270376, -1.7551165719633275, -2.074100961530956, -2.0116304022964684, -1.5886118784948984, -0.8949302981956571, -0.054581596036655355, 0.8058811105655721, 1.5704763097457288, 2.1640265638063596, 2.5575770857165523, 2.761281977154802, 2.8131185718556893, 2.7535769001690653, 2.6132374116023556, 2.41852549318736, 2.2004599395092086, 1.988999759195778, 1.812187197388191, 1.712122020559491, 1.7363699292335113, 1.9183278121911513, 2.2738257937121773, 2.7870423868286807, 3.402456505289315, 4.047515420096644, 4.648775603954967, 5.147464189108305, 5.530199586772476, 5.833529038206159, 6.134652521396426, 6.539535562900241, 7.155848332639302, 8.070414668946668, 9.328943628471677, 10.918281314615967, 12.785605556147363, 14.866423116470724, 17.107891188203872, 19.498580292076078, 22.074317143711664, 24.919899705625653, 28.157440368003503, 31.9097956946241, 36.275166698245435, 41.304973358816454, 46.97883507698724, 53.205287100068524, 59.82969788487038, 66.64087722867654, 73.40779884607333, 79.91821588168855, 86.00752753262773, 91.60064809653764, 96.75188915477419, 101.66743661587006, 106.70460796103863, 112.3156072405998, 118.94018764853767, 126.88071725247491, 136.15562714935854, 146.37302292018552, 156.68155375606483, 165.81275793573548, 172.24174731707524, 174.46892203836632, 171.34982970233142, 162.38943409454515, 147.9516925299859, 129.34064868357336, 108.66566564234145, 88.51287702423652, 71.54116976220826, 60.018884545134405, 55.40767827978098, 58.14705300061065, 67.62348360129519, 82.31273035031066, 100.12115849129016, 118.79252871484319, 136.2739962892324, 151.02074953128727, 162.14620535359873, 169.40269365839498, 173.04742840577512, 173.63540540150913, 171.80748973121885, 168.12419673941935, 162.97380339022595, 156.58019993140687, 149.06057334442724, 140.49938542346416, 131.03047868728135, 120.88018810896922, 110.36645255841222, 99.8590736632206, 89.71973940397402, 80.24425952165575, 71.61697124849918, 63.89863145863566, 57.04279791836636, 50.926176583044985, 45.39428111606999, 40.29962836918817, 35.52517892432068, 31.004546466986596, 26.727681107966106, 22.72791634112363, 19.05733547804288, 15.76824660203588, 12.896805929990485, 10.439146808736961, 8.343608705949277, 6.518301665555141, 4.842720131859084, 3.19350929078696, 1.4743260500651258, -0.3630208683470837, -2.3169585137799777, -4.331800967907609, -6.297621526969359, -8.083507212508165, -9.5758546464229, -10.70175190004283, -11.43684319605934, -11.805624338351091, -11.876071789456802, -11.75600082646371, -11.569958462048822, -11.425293072890906, -11.401912484793211, -11.552607355420465, -11.904801229696115, -12.459281939905711, -13.195308729901553, -14.08017115754382, -15.070266205866737, -16.10721631437246, -17.133749550004634, -18.091965400911693, -18.90254817549151, -19.48472515734146, -19.780671869455727, -19.762206208696192, -19.434228638774012, -18.836022358724346, -18.037486895702195, -17.130639259434474, -16.211401357666713, -15.345516298446267, -14.560428186924335, -13.862779152643615, -13.233405348596127, -12.638313084973134, -12.060959861439803, -11.505826259899411, -10.996221202859427, -10.57201197501543, -10.273576989127381, -10.126965713260306, -10.123618543137269, -10.214532371187227, -10.325166664365499, -10.369206031478202, -10.269816881773657, -9.978075766140728, -9.48667722154062, -8.835377837567348, -8.110762434329587, -7.427137545133081, -6.889444150286735, -6.576048158291635, -6.534974120596583, -6.775127611523702, -7.253248823151033, -7.885063852425014, -8.574998606380312, -9.239484838672864, -9.81795343597639, -10.268523178139327, -10.570211750249543, -10.734359053126774, -10.794653493124017, -10.780597140623197, -10.720890945952343, -10.651603387439392, -10.597216984559031, -10.563531523062537, -10.558407507221972, -10.60471251965382, -10.721262726987103, -10.913596620415007, -11.180414648848739, -11.511685839845594, -11.882122075787773, -12.24396075588322, -12.538139842123886, -12.713382227672625, -12.729444550062146, -12.563010469749287, -12.225439761479489, -11.764838205091637, -11.238571389052538, -10.700946057889144, -10.204058149971942, -9.778125792157056, -9.422395383314628, -9.108564840290036, -8.791549344352264, -8.42985733313703, -7.996221708485883, -7.481529498489944, -6.890918342749518, -6.234796394592002, -5.526533144118856, -4.773132769378386, -3.9738671812390205, -3.13605445313196, -2.305770505655736, -1.5933094615791155, -1.162511280513114, -1.2088806695673568, -1.9091974351101024, -3.33712248032913, -5.3742248547907625, -7.639465647542465, -9.4769052323094, -10.009955641208647, -8.260339831638246, -3.3178383695456386, 5.459203485947884, 18.25714332341031, 34.69671223366966, 53.823771687042324, 74.19974849020429, 94.06998629194288, 111.60668455201537, 125.18786149671595, 133.62064552889413, 136.28251151628456, 133.1782674406399, 124.88595375052785, 112.42754951601276, 97.08863231884405, 80.21018703218603, 63.026258410623356, 46.55992098928846, 31.558666319204736, 18.487188883810205, 7.574967543561163, -1.1290673077549278, -7.699420687583913, -12.290602897454782, -15.11802800841009, -16.438670314594734, -16.54921920582092, -15.77572134138182, -14.453052630173747, -12.910426246647424, -11.436303128263107, -10.253260759508269, 